vi "UHR-Fleezers Control (host) - 10.8MV_trial.vi"() -> ()   [LabVIEW 2010] (continued)
          }
          frame #2 {
            n1089 = property on="Green Laser ON/Interlacing" class="Bool (strict)"("Val(Sgnl)"=TRUE ("Value (Signaling)")) -> ()  [unwired: 2 in, 2 out]
            n1090 = property on="Flip Green Filter" class="Bool (strict)"("Val(Sgnl)"=TRUE ("Value (Signaling)")) -> ()  [unwired: 2 in, 2 out]
            n1091 = property on="Green laser mode" class="RadioBtnsControl (strict)"("Val(Sgnl)"=enum32{"Laser ON", "Laser OFF", "Interlace"}."Laser ON" ("Value (Signaling)")) -> ()  [unwired: 2 in, 2 out]
          }
          frame #3 {
            n1092 = Wait (ms)(milliseconds to wait=u32 500) -> ()  [unwired: 1 out]
          }
          frame #4 {
            n1093 = property on="Confocal Image" class="Bool (strict)"("Val(Sgnl)"=TRUE ("Value (Signaling)")) -> ()  [unwired: 2 in, 2 out]
          }
          frame #5 {
            n1094 = Wait (ms)(milliseconds to wait=u32 2000) -> ()  [unwired: 1 out]
          }
          frame #6 {
            n1095 = while {
              stop <- w5166 stop-if-true
              n1096 = local read "Saving..."() -> (w5167:bool)
              n1097 = Not(x=w5167) -> (.not. x?=w5166:bool)
            }
          }
          frame #7 {
            n1098 = property on="Flip Green Filter" class="Bool (strict)"("Val(Sgnl)"=TRUE ("Value (Signaling)")) -> ()  [unwired: 2 in, 2 out]
            n1099 = property on="Green Laser ON/Interlacing" class="Bool (strict)"("Val(Sgnl)"=w5171) -> ()  [unwired: 2 in, 2 out]
            n1100 = property on="Green laser mode" class="RadioBtnsControl (strict)"("Val(Sgnl)"=w5170) -> ()  [unwired: 2 in, 2 out]
          }
          frame #8 {
            n1101 = property on="Green FB On/Off" class="Bool (strict)"("Val(Sgnl)"=w5172) -> ()  [unwired: 2 in, 2 out]
          }
        }
      }
      event "Stop All": Value Change {
        n1102 = event-data() -> ()  [unwired: 1 in, 5 out]
        n1103 = local read "Stop All"() -> (w5173:bool)
      }
    }
    n1104 = node-c288() -> ()  [unwired: 1 in, 1 out]
  }
  n1105 = node-c288() -> (w76:T26)  [unwired: 4 out]
  n1106 = timed-loop "Mouse control: trap position (AOM deflection), set confocal spot from image" {
    tunnel: [w5175] -> w34
    tunnel: w24 -> [w5174]
    timing: w76 -> [_]
    timing-out: [_] -> w75
    stop <- w5175 stop-if-true
    n1107 = node-c288() -> ()  [unwired: 2 out]
    n1108 = event shown="[0] \"Pane\": Mouse Down" {
      selector: _ -> [_ _]
      dyn-events: _ -> [_ _]
      timeout: _ -> [_ _]
      tunnel: w5174 -> [w5178 _]
      event Mouse Down {
        n1109 = event-data() -> ("Time"=w5180:u32, "Coords"=w5179:T7, "Button"=w5181:u16)  [unwired: 6 out]
        n1110 = case shown="1" w5181 {
          tunnel: w5180 -> [_ _ w5284]
          tunnel: w5179 -> [_ w5218 w5282]
          tunnel: w5178 -> [_ _ w5280]
          frame 0, Default {
          }
          frame 1 {
            n1111 = property on="APD 2" class="ImageControl"() -> ("Displayed Image Position"=w5188:cluster{"Left":i32, "Top":i32})  [unwired: 2 in, 2 out]
            n1112 = property on="APD 1" class="ImageControl"() -> ("Displayed Image Position"=w5217:cluster{"Left":i32, "Top":i32})  [unwired: 2 in, 2 out]
            n1113 = property on="Detection Laser X" class="ImageControl"() -> ("Displayed Image Position"=w5214:cluster{"Left":i32, "Top":i32})  [unwired: 2 in, 2 out]
            n1114 = property on="Detection Laser Y" class="ImageControl"() -> ("Displayed Image Position"=w5213:cluster{"Left":i32, "Top":i32})  [unwired: 2 in, 2 out]
            n1115 = property on="APD 2" class="ImageControl"() -> ("Displayed Image Size"=w5187:cluster{"Width":u32, "Height":u32})  [unwired: 2 in, 2 out]
            n1116 = property on="APD 1" class="ImageControl"() -> ("Displayed Image Size"=w5215:cluster{"Width":u32, "Height":u32})  [unwired: 2 in, 2 out]
            n1117 = property on="Detection Laser X" class="ImageControl"() -> ("Displayed Image Size"=w5216:cluster{"Width":u32, "Height":u32})  [unwired: 2 in, 2 out]
            n1118 = property on="Detection Laser Y" class="ImageControl"() -> ("Displayed Image Size"=w5212:cluster{"Width":u32, "Height":u32})  [unwired: 2 in, 2 out]
            n1119 = Unbundle By Name(w5187) -> ("Width"=w5184:u32, "Height"=w5183:u32)
            n1120 = Unbundle By Name(w5188) -> ("Left"=w5186:i32, "Top"=w5185:i32)
            n1121 = Unbundle By Name(w5215) -> ("Width"=w5209:u32, "Height"=w5208:u32)
            n1122 = Unbundle By Name(w5216) -> ("Width"=w5205:u32, "Height"=w5204:u32)
            n1123 = Unbundle By Name(w5212) -> ("Width"=w5201:u32, "Height"=w5200:u32)
            n1124 = Unbundle By Name(w5217) -> ("Left"=w5211:i32, "Top"=w5210:i32)
            n1125 = Unbundle By Name(w5214) -> ("Left"=w5207:i32, "Top"=w5206:i32)
            n1126 = Unbundle By Name(w5213) -> ("Left"=w5203:i32, "Top"=w5202:i32)
            n1127 = Bundle("Left"=w5186, "Top"=w5185, "Width"=w5184, "Height"=w5183) -> (w5182:T35)  [unwired: 1 in]
            n1128 = Bundle("Left"=w5211, "Top"=w5210, "Width"=w5209, "Height"=w5208) -> (w5199:T35)  [unwired: 1 in]
            n1129 = Bundle("Left"=w5207, "Top"=w5206, "Width"=w5205, "Height"=w5204) -> (w5198:T35)  [unwired: 1 in]
            n1130 = Bundle("Left"=w5203, "Top"=w5202, "Width"=w5201, "Height"=w5200) -> (w5197:T35)  [unwired: 1 in]
            n1131 = Build Cluster Array(w5182, w5199, w5198, w5197) -> (w5196:T36)
            n1132 = for {
              tunnel: w5218 -> [w5229]
              tunnel: w5196 -> [w5230] mode=indexing
              shift-right: [w5227] -> w5194
              shift-left: TRUE -> [w5228]
              shift-right: [w5226] -> w5192
              shift-left: _ -> [w5222]
              shift-right: [w5225] -> w5191
              shift-left: _ -> [w5221]
              shift-right: [w5224] -> w5190
              shift-left: _ -> [w5220]
              shift-right: [w5223] -> w5189
              shift-left: _ -> [w5219]
              n1133 = case shown="True" w5228 {
                selector: w5228 -> [w5235 _]
                tunnel: w5230 -> [_ w5244]
                tunnel: w5229 -> [_ w5242]
                tunnel: [w5235 w5240] -> w5227
                tunnel: [w5234 w5239] -> w5226
                tunnel: [w5233 w5238] -> w5225
                tunnel: [w5232 w5237] -> w5224
                tunnel: [w5231 w5236] -> w5223
                tunnel: w5222 -> [w5234 _]
                tunnel: w5221 -> [w5233 _]
                tunnel: w5220 -> [w5232 _]
                tunnel: w5219 -> [w5231 _]
                frame False {
                }
                frame True {
                  n1134 = Unbundle(w5244) -> (w5243:T35)
                  n1135 = call "isclickinwindow.vi"("Image Param"=w5243, "Point32"=w5242) -> ("4 Y"=w5236:i32, "3 Height"=w5237:i32, "2 X"=w5238:i32, "1 Width"=w5239:i32, "In image?"=w5241:bool)  [unwired: 1 in]
                  n1136 = Not(x=w5241) -> (.not. x?=w5240:bool)
                }
              }
            }
            n1137 = Not(x=w5194) -> (.not. x?=w5193:bool)
            n1138 = case shown="True" w5193 {
              tunnel: w5191 -> [_ w5257]
              tunnel: w5189 -> [_ w5256]
              tunnel: w5192 -> [_ w5255]
              tunnel: w5190 -> [_ w5254]
              frame False {
              }
              frame True {
                w5250 = FALSE ("Get Point")
                n1139 = local read "Scan lines (y)"() -> (w5259:u64)
                n1140 = local read "Actual MCL Inc (V)"() -> (w5251:dbl)
                n1141 = local read "Scan steps (MCL)"() -> (w5258:u64)
                n1142 = Divide "Y Pix/step"(x=w5254, y=w5259) -> (x/y=w5266:dbl)
                n1143 = Divide "Y V/pix"(x=w5251, y=w5266) -> (x/y=w5265:dbl)
                n1144 = Divide "Y half step offset"(x=w5251, y=2.0) -> (x/y=w5267:dbl)
                n1145 = Divide "X pix/step"(x=w5255, y=w5258) -> (x/y=w5264:dbl)
                n1146 = Negate(x=w5267) -> (-x=w5268:dbl)
                n1147 = local read "Initial Y"() -> (w5274:dbl)
                n1148 = Multiply(x=w5256, y=w5265) -> (x*y=w5275:dbl)
                n1149 = Divide "X half step offset"(x=w5251, y=2.0) -> (x/y=w5261:dbl)
                n1150 = Divide "X V/pix"(x=w5251, y=w5264) -> (x/y=w5263:dbl)
                n1151 = Multiply(x=w5251, y=w5258) -> (x*y=w5270:dbl)
                n1152 = Compound Arithmetic op=ADD(w5268, w5275, w5274) -> (w5252:dbl)
                "Pointer Y (V)" <- w5252
                n1153 = Multiply(x=w5263, y=w5257) -> (x*y=w5272:dbl)
                n1154 = Negate(x=w5261) -> (-x=w5260:dbl)
                n1155 = local read "Initial X"() -> (w5273:dbl)
                n1156 = Negate(x=w5272) -> (-x=w5271:dbl)
                n1157 = Compound Arithmetic op=ADD(w5260, w5270, w5273, w5271) -> (w5253:dbl)
                "Pointer X (V)" <- w5253
                n1158 = Or(x="Set X Only", y="Set Confocal Spot (X-Y)") -> (x .or. y?=w5246:bool)
                n1159 = Or(x="Set Confocal Spot (X-Y)", y="Set Y Only") -> (x .or. y?=w5245:bool)
                n1160 = case shown="True" w5246 {
                  tunnel: w5253 -> [_ w5276]
                  frame False {
                  }
                  frame True {
                    n1161 = property on="AO2" class="Slide (strict)"("Val(Sgnl)"=w5276) -> ()  [unwired: 2 in, 2 out]
                  }
                }
                n1162 = case shown="True" w5245 {
                  tunnel: w5252 -> [_ w5277]
                  frame False {
                  }
                  frame True {
                    n1163 = property on="AO1" class="Slide (strict)"("Val(Sgnl)"=w5277) -> ()  [unwired: 2 in, 2 out]
                  }
                }
                n1164 = local write "Set Confocal Spot (X-Y)"(w5250) -> ()
                n1165 = local write "Set X Only"(w5250) -> ()
                n1166 = local write "Set Y Only"(w5250) -> ()
              }
            }
          }
          frame 3 {
            n1167 = local read "BD 2 Frequency 1 (MHz)"() -> (w5278:dbl)
            n1168 = local read "BD 1 Frequency 1 (MHz)"() -> (w5279:dbl)
            n1169 = local write "Manipulating Trap"(TRUE ("Manipulating Trap")) -> ()
            n1170 = local write "Coords"(T7 {"Horizontal"=0, "Vertical"=0} ("Coords")) -> ()
            n1171 = while {
              tunnel: w5284 -> [w5289]
              tunnel: w5282 -> [w5288]
              tunnel: w5280 -> [w5287]
              tunnel: w5279 -> [w5286]
              tunnel: w5278 -> [w5285]
              stop <- w5290 stop-if-true
              n1172 = event shown="[0] \"Pane\": Mouse Move" {
                selector: _ -> [_ _]
                dyn-events: _ -> [_ _]
                timeout: _ -> [_ _]
                tunnel: ["Force Manip Abort" w5354] -> w5290
                tunnel: w5289 -> [w5297 _]
                tunnel: w5288 -> [w5295 _]
                tunnel: w5287 -> [w5294 _]
                tunnel: w5286 -> [w5293 _]
                tunnel: w5285 -> [w5292 _]
                event Mouse Move {
                  n1173 = event-data() -> ("Time"=w5298:u32, "Coords"=w5299:T7)  [unwired: 3 out]
                  n1174 = Less?(x=w5298, y=w5297) -> (x < y?=w5296:bool)
                  n1175 = case "Makes sure old motion events prior to mouse click aren't used" shown="False" w5296 {
                    tunnel: w5299 -> [w5341 _]
                    tunnel: w5295 -> [w5342 _]
                    tunnel: w5294 -> [w5319 _]
                    tunnel: w5293 -> [w5315 _]
                    tunnel: w5292 -> [w5314 _]
                    frame False {
                      n1176 = Subtract(x=w5341, y=w5342) -> (x-y=w5340:T7)
                      "Coords" <- w5340
                      n1177 = local read "Y RF Frequency Limits (MHz)"() -> (w5300:T16)
                      n1178 = To Double Precision Float(number=w5340) -> (double precision float=w5339:cluster{"Horizontal":dbl, "Vertical":dbl})
                      n1179 = Multiply(x=cluster{"Horizontal":dbl, "Vertical":dbl} {"Horizontal"=-1.0, "Vertical"=1.0}, y="Manipulation Scaling") -> (x*y=w5335:cluster{"Horizontal":dbl, "Vertical":dbl})
                      n1180 = local read "X RF Frequency Limits (MHz)"() -> (w5301:T16)
                      n1181 = Multiply(x=w5339, y=w5335) -> (x*y=w5337:cluster{"Horizontal":dbl, "Vertical":dbl})
                      n1182 = Unbundle By Name(w5337) -> ("Horizontal"=w5332:dbl, "Vertical"=w5336:dbl)
                      n1183 = Unbundle By Name(w5300) -> ("Maximum"=w5303:dbl, "Minimum"=w5302:dbl)
                      n1184 = Boolean To (0,1)(Boolean="Manip. X?") -> (0, 1=w5330:i16)
                      n1185 = Boolean To (0,1)(Boolean="Manip. Y?") -> (0, 1=w5327:i16)
                      n1186 = local read "BD 1 Frequency 2 (MHz)"() -> (w5317:dbl)
                      n1187 = Multiply(x=w5336, y=w5327) -> (x*y=w5329:dbl)
                      n1188 = Multiply(x=w5330, y=w5332) -> (x*y=w5333:dbl)
                      n1189 = local read "BD 2 Frequency 2 (MHz)"() -> (w5316:dbl)
                      n1190 = Unbundle By Name(w5301) -> ("Maximum"=w5305:dbl, "Minimum"=w5304:dbl)
                      n1191 = Add(x=w5314, y=w5329) -> (x+y=w5307:dbl)
                      n1192 = Add(x=w5315, y=w5333) -> (x+y=w5309:dbl)
                      n1193 = In Range and Coerce(upper limit=w5305, x=w5309, lower limit=w5304) -> (coerced(x)=w5308:dbl)  [unwired: 1 out]
                      n1194 = In Range and Coerce(upper limit=w5303, x=w5307, lower limit=w5302) -> (coerced(x)=w5306:dbl)  [unwired: 1 out]
                      n1195 = Subtract(x=w5308, y=w5317) -> (x-y=w5326:dbl)
                      n1196 = Subtract(x=w5306, y=w5316) -> (x-y=w5325:dbl)
                      n1197 = Square(x=w5326) -> (x^2=w5324:dbl)
                      n1198 = Square(x=w5325) -> (x^2=w5323:dbl)
                      n1199 = Add(x=w5324, y=w5323) -> (x+y=w5322:dbl)
                      n1200 = Square Root(x=w5322) -> (sqrt(x)=w5318:dbl)
                      n1201 = In Range and Coerce(upper limit="Limit Max (MHz)", x=w5318, lower limit="Limit Min (MHz)") -> (In Range?=w5311:bool)  [unwired: 1 out]
                      n1202 = Not(x="Limits Enable") -> (.not. x?=w5310:bool)
                      n1203 = Or(x=w5311, y=w5310) -> (x .or. y?=w5312:bool)
                      n1204 = case shown="True" w5312 {
                        tunnel: w5319 -> [_ w5352]
                        tunnel: w5318 -> [_ w5343]
                        tunnel: w5308 -> [_ w5350]
                        tunnel: w5317 -> [_ w5349]
                        tunnel: w5306 -> [_ w5348]
                        tunnel: w5316 -> [_ w5347]
                        tunnel: w5301 -> [_ w5345]
                        tunnel: w5300 -> [_ w5344]
                        frame False {
                        }
                        frame True {
                          n1205 = local read "BD 1 Frequency 3 (MHz)"() -> (w5351:dbl)
                          n1206 = local read "BD 2 Frequency 3 (MHz)"() -> (w5346:dbl)
                          n1207 = local write "Trap Delta (MHz)"(w5343) -> ()
                          n1208 = property on="Initial delta (MHz)" class="DigNum (strict)"("Val(Sgnl)"=w5343) -> ()  [unwired: 2 in, 2 out]
                          n1209 = call "set RF board frequency - interlace.vi"("Board 2 Frequency Limits"=w5344, "Board 1 Frequency Limits"=w5345, "FPGA VI Reference In"=w5352, "Board 2 Frequency 3 (MHz)"=w5346, "Board 1 Frequency 3 (MHz)"=w5351, "Board 2 Frequency 2 (MHz)"=w5347, "Board 2 Frequency 1 (MHz)"=w5348, "Board 1 Frequency 2 (MHz)"=w5349, "Board 1 Frequency 1  (MHz)"=w5350) -> ()  [unwired: 1 in, 2 out]
                          n1210 = local write "BD 2 Frequency 1 (MHz)"(w5348) -> ()
                          n1211 = local write "BD 1 Frequency 1 (MHz)"(w5350) -> ()
                        }
                      }
                    }
                    frame True {
                    }
                  }
                }
                event Mouse Up {
                  n1212 = event-data() -> ("Button"=w5353:u16)  [unwired: 8 out]
                  n1213 = case shown="3" w5353 {
                    tunnel: [FALSE TRUE] -> w5354
                    frame 0, Default {
                    }
                    frame 3 {
                      n1214 = local write "Manipulating Trap"(FALSE ("Manipulating Trap")) -> ()
                    }
                  }
                }
              }
            }
          }
        }
      }
      event Mouse Move {
        n1215 = event-data() -> ()  [unwired: 6 out]
      }
    }
    n1216 = local read "Stop All"() -> (w5175:bool)
    n1217 = node-c288() -> ()  [unwired: 2 out]
  }
  n1218 = node-c288(i64 1 ("Period"), 1 ("Processor")) -> (w164:T26)  [unwired: 2 out]
  n1219 = timed-loop "Acquire Data" {
    tunnel: w24 -> [w5612]
    tunnel: w40 -> [w5611]
    tunnel: [w5642] -> w33
    tunnel: [w5636] -> w32
    timing: w164 -> [_]
    timing-out: [_] -> w163
    tunnel: w59 -> [w5440]
    stop <- "Stop All" stop-if-true
    (unwired) u32 0 ("Number of Elements")
    w5427 = "NI_ChannelName" ("name")
    n1220 = node-c288() -> ()  [unwired: 2 out]
    n1221 = First Call?() -> (First Call?: T/F=w5393:bool)
    n1222 = Or(x="Reset", y=w5393) -> (x .or. y?=w5394:bool)
    n1223 = case "Reset data stream" shown="True" w5394 {
      tunnel: w5612 -> [w5730 w5738]
      tunnel: w5611 -> [w5729 w5737]
      tunnel: [w5730 w5732] -> w5607
      tunnel: [w5729 w5731] -> w5606
      frame False {
      }
      frame True {
        w5735 = TRUE ("AI to FIFO")
        n1224 = local write "Overflow (data lost)"(FALSE ("Overflow (data lost)")) -> ()
        n1225 = call "reset FPGA DMA.vi"("error in"=w5737, "FPGA VI Reference In"=w5738) -> ("error out"=w5733:errorcluster, "FPGA VI Reference Out"=w5734:T19)
        n1226 = xnode "Read/Write Control"("FPGA VI Reference In"=w5734, "error in"=w5733, "AI to FIFO"=w5735, "APD to FIFO"=w5735) -> ("FPGA VI Reference Out"=w5732:T19, "error out"=w5731:errorcluster)
      }
    }
    n1227 = Or(x="Start AOD Scan", y="Trap Raster Scan") -> (x .or. y?=w5557:bool)
    n1228 = case "Start AOM raster scan" shown="True" w5557 {
      tunnel: w5607 -> [w7338 w7348]
      tunnel: w5606 -> [w7337 w7347]
      tunnel: [w7338 w7341] -> w5605
      tunnel: [w7337 w7340] -> w5604
      frame False {
      }
      frame True {
        n1229 = case shown="True" "Restart DMA? (AOD)" {
          tunnel: [w7759 w7761] -> w7342
          tunnel: [w7758 w7760] -> w7343
          tunnel: w7348 -> [w7759 w7763]
          tunnel: w7347 -> [w7758 w7762]
          frame False {
          }
          frame True {
            n1230 = local write "Overflow (data lost)"(FALSE ("Overflow (data lost)")) -> ()
            n1231 = call "reset FPGA DMA.vi"("error in"=w7762, "FPGA VI Reference In"=w7763) -> ("error out"=w7760:errorcluster, "FPGA VI Reference Out"=w7761:T19)
          }
        }
        n1232 = local write "Trap Raster Scan"(FALSE ("Trap Raster Scan")) -> ()
        n1233 = case shown="False" "Move MCL Also?" {
          tunnel: w7343 -> [w7351 w7460]
          tunnel: w7342 -> [w7352 w7461]
          tunnel: [w7350 w7464] -> w7341
          tunnel: [w7349 w7463] -> w7340
          frame False {
            w7353 = TRUE ("AI to FIFO")
            n1234 = xnode "Read/Write Control"("FPGA VI Reference In"=w7352, "error in"=w7351, "AI to FIFO"=w7353, "APD to FIFO"=w7353, "Start scan"=w7353) -> ("FPGA VI Reference Out"=w7350:T19, "error out"=w7349:errorcluster)
          }
          frame True {
            w7457 = FALSE ("1D or 2D Scan?")
            w7462 = TRUE ("AI to FIFO")
            # "Count for MCL loop"
            # "N total cycles"
            # "N steps"
            # "V_int"
            n1235 = local read "Scan Range (nm)"() -> (w7439:dbl)
            n1236 = local read "Number of F/B Scans (AOD)"() -> (w7456:u16)
            n1237 = Sign(1:w7439) -> (0:w7438:dbl)
            n1238 = Compound Arithmetic op=MULTIPLY(w7439, "MCL Step Position Ratio", "MCL/AOM Scale Tweak") -> (w7443:dbl)
            n1239 = Negate(x=w7438) -> (-x=w7435:dbl)
            n1240 = Multiply(x=w7435, y="MCL Step Increment (V_int)") -> (x*y=w7437:dbl)
            n1241 = Divide(x=w7443, y="MCL X Cal (nm/V)") -> (x/y=w7449:dbl)
            n1242 = Multiply(x=32767.0 ("y"), y=w7449) -> (x*y=w7455:dbl)
            n1243 = local read "Total Counts (ticks)"() -> (w7440:u32)
            n1244 = local read "Cycles/step (AOD)"() -> (w7451:u64)
            n1245 = local read "Scan steps (AOD)"() -> (w7452:u64)
            n1246 = Divide(x=w7455, y=10.0) -> (x/y=w7448:dbl)
            n1247 = Divide(x=w7448, y="MCL Step Increment (V_int)") -> (x/y=w7446:dbl)
            n1248 = Absolute Value(x=w7446) -> (abs(x)=w7434:dbl)
            n1249 = Compound Arithmetic op=MULTIPLY(w7452, w7451, w7440) -> (w7447:u64)
            n1250 = local write "wait to reset values"(w7462) -> ()
            n1251 = local write "MCL Scanning"(w7462) -> ()
            n1252 = Divide(x=w7447, y=w7434) -> (x/y=w7444:dbl)
            "MCL Count" <- w7444
            n1253 = xnode "Read/Write Control"("FPGA VI Reference In"=w7461, "error in"=w7460, "Scan steps (MCL)"=w7434, "Number of scans (MCL)"=w7456, "Cycles per step (MCL)"=u64 1, "Scan freq.  increment (MCL)"=w7437, "1D or 2D Scan?"=w7457, "MCL Scan Axis"=w7457, "Cont. Scan (MCL)"=w7457, "MCL count"=w7444) -> ("FPGA VI Reference Out"=w7459:T19, "error out"=w7458:errorcluster)
            n1254 = xnode "Read/Write Control"("FPGA VI Reference In"=w7459, "error in"=w7458, "AI to FIFO"=w7462, "APD to FIFO"=w7462, "Start scan"=w7462, "Start scan (MCL)"=w7462) -> ("FPGA VI Reference Out"=w7464:T19, "error out"=w7463:errorcluster)
          }
        }
        "Raster Scanning..." <- TRUE ("Scanning...")
      }
    }
    n1255 = And(x="Save scans", y=w5557) -> (x .and. y?=w5603:bool)
    n1256 = Compound Arithmetic op=OR("Start MCL Scan", "Confocal Image", "Confocal Linescan") -> (w5555:bool)
    n1257 = And(x="Save Data (MCL)", y=w5555) -> (x .and. y?=w5602:bool)
    n1258 = case "Start MCL raster scan" shown="True" w5555 {
      tunnel: w5605 -> [w6615 w6630]
      tunnel: w5604 -> [w6614 w6629]
      tunnel: [w6615 w6625] -> w5362
      tunnel: [w6614 w6624] -> w5361
      tunnel: [FALSE w6623] -> w5588
      tunnel: "Start MCL Scan" -> [_ w6618]
      tunnel: "Confocal Image" -> [_ w6617]
      tunnel: "Confocal Linescan" -> [_ _]
      frame False {
      }
      frame True {
        w6623 = TRUE
        n1259 = case shown="True" "Restart DMA? (MCL)" {
          tunnel: [w6875 w6877] -> w6628
          tunnel: [w6874 w6876] -> w6627
          tunnel: w6630 -> [w6875 w6880]
          tunnel: w6629 -> [w6874 w6879]
          frame False {
          }
          frame True {
            n1260 = call "reset FPGA DMA.vi"("error in"=w6879, "FPGA VI Reference In"=w6880) -> ("error out"=w6876:errorcluster, "FPGA VI Reference Out"=w6877:T19)
            n1261 = local write "Overflow (data lost)"(FALSE ("Overflow (data lost)")) -> ()
          }
        }
        n1262 = case shown="False" w6618 {
          selector: w6618 -> [_ w6634]
          tunnel: w6617 -> [w6633 _]
          tunnel: [w6633 w6634] -> w6616
          frame False {
            n1263 = property on="2D or 1D Scan" class="Bool (strict)"("Val(Sgnl)"=w6633) -> ()  [unwired: 2 in, 2 out]
            n1264 = property on="Confocal Image" class="Bool (strict)"("Value"=FALSE ("Start Confocal Map")) -> ()  [unwired: 2 in, 2 out]
          }
          frame True {
          }
        }
        n1265 = local write "MCL Scanning"(w6623) -> ()
        n1266 = local read "AO1"() -> (w6620:dbl)
        n1267 = local read "AO2"() -> (w6619:dbl)
        n1268 = case shown="True" "Center Scan" {
          tunnel: w6628 -> [w6641 w6753]
          tunnel: w6627 -> [w6640 w6752]
          tunnel: [w6639 w6751] -> w6625
          tunnel: [w6638 w6750] -> w6624
          tunnel: [w6636 w6737] -> w6622
          tunnel: [w6635 w6736] -> w6621
          tunnel: w6620 -> [w6636 w6742]
          tunnel: w6619 -> [w6635 w6745]
          tunnel: w6616 -> [_ _]
          frame False {
            w6637 = TRUE ("AI to FIFO")
            n1269 = xnode "Read/Write Control"("FPGA VI Reference In"=w6641, "error in"=w6640, "AI to FIFO"=w6637, "APD to FIFO"=w6637, "Start scan (MCL)"=w6637) -> ("FPGA VI Reference Out"=w6639:T19, "error out"=w6638:errorcluster)
          }
          frame True {
            w6749 = TRUE ("AI to FIFO")
            n1270 = local read "Scan steps (MCL)"() -> (w6728:u64)
            n1271 = local read "Scan lines (y)"() -> (w6724:u64)
            n1272 = local read "Fast Scan Dir"() -> (w6735:bool)
            n1273 = local read "Actual MCL Inc (V)"() -> (w6725:dbl)
            n1274 = Decrement(x=w6724) -> (x-1=w6723:u64)
            n1275 = Decrement(x=w6728) -> (x-1=w6727:u64)
            n1276 = Multiply(x=w6725, y=w6723) -> (x*y=w6722:dbl)
            n1277 = Divide(x=w6722, y=2.0) -> (x/y=w6732:dbl)
            n1278 = Multiply(x=w6725, y=w6727) -> (x*y=w6726:dbl)
            n1279 = Divide(x=w6726, y=2.0) -> (x/y=w6731:dbl)
            n1280 = Select(t=w6731, s=w6735, f=w6732) -> (s? t:f=w6730:dbl)
            n1281 = Select(t=w6732, s=w6735, f=w6731) -> (s? t:f=w6734:dbl)
            n1282 = Subtract(x=w6742, y=w6734) -> (x-y=w6733:dbl)
            n1283 = Subtract(x=w6745, y=w6730) -> (x-y=w6729:dbl)
            n1284 = local read "2D or 1D Scan"() -> (w6747:bool)
            n1285 = Not(x=w6735) -> (.not. x?=w6741:bool)
            n1286 = Not(x=w6747) -> (.not. x?=w6743:bool)
            n1287 = And(x=w6735, y=w6743) -> (x .and. y?=w6744:bool)
            n1288 = And(x=w6743, y=w6741) -> (x .and. y?=w6746:bool)
            n1289 = Select(t=w6745, s=w6746, f=w6729) -> (s? t:f=w6736:dbl)
            n1290 = Select(t=w6742, s=w6744, f=w6733) -> (s? t:f=w6737:dbl)
            n1291 = call "Volt to I16.vi"("Voltage In"=w6737) -> ("I16 Voltage Out"=w6740:i16)
            n1292 = call "Volt to I16.vi"("Voltage In"=w6736) -> ("I16 Voltage Out"=w6739:i16)
            n1293 = xnode "Read/Write Control"("FPGA VI Reference In"=w6753, "error in"=w6752, "AI to FIFO"=w6749, "APD to FIFO"=w6749, "Start scan (MCL)"=w6749, "AO1"=w6740, "AO2"=w6739) -> ("FPGA VI Reference Out"=w6751:T19, "error out"=w6750:errorcluster)
          }
        }
        "Initial Y" <- w6622
        "Initial X" <- w6621
        "wait to reset values" <- w6623
      }
    }
    n1294 = local read "Trap Pos Elements/DMA read"() -> (w5436:u32)
    n1295 = local read "Trap AI Elements/DMA read"() -> (w5360:u32)
    n1296 = local read "APD Elements/DMA read"() -> (w5479:u32)
    n1297 = local read "Trap AI FIFO Depth"() -> (w5652:u32)
    n1298 = xnode "Invoke Method"("FPGA VI Reference In"=w5362, "error in"=w5361, "Number of Elements"=w5436, "Timeout (ms)"=-1) -> ("Data"=w5400:u16[], "Elements Remaining"=→"Trap Pos FIFO El Remaining":u32)  [unwired: 2 out]
    n1299 = xnode "Invoke Method"("FPGA VI Reference In"=w5362, "error in"=w5361, "Number of Elements"=w5360, "Timeout (ms)"=-1 ("Timeout")) -> ("FPGA VI Reference Out"=w5364:T19, "error out"=w5363:errorcluster, "Data"=w5359:i16[], "Elements Remaining"=w5365:u32)
    "Trap AI FIFO El. Rem." <- w5365
    n1300 = xnode "Get APD Data"("FPGA VI Reference In"=w5362, "error in"=w5361, "Number of Elements"=w5479, "Timeout (ms)"=-1) -> ("Data"=w5478:u32[], "Elements Remaining"=→"APD FIFO Elements Remaining":u32)  [unwired: 2 out]
    n1301 = Subtract(x=w5652, y=w5360) -> (x-y=w5651:u32)
    n1302 = Decimate 1D Array(w5400) -> (w5397:u16[], w5399:u16[], w5398:u16[])
    n1303 = Divide(x=w5365, y=w5651) -> (x/y=w5650:dbl)
    "Buffer Status" <- w5650
    n1304 = To Unsigned Long Integer(number=w5397) -> (unsigned 32bit integer=w5396:u32[])
    n1305 = Join Numbers(hi=w5399, lo=w5398) -> ((hi.lo)=w5395:u32[])
    n1306 = Equal?(x=w5650, y=1.0) -> (x = y?=w5648:bool)
    n1307 = Join Numbers(hi=w5396, lo=w5395) -> ((hi.lo)=w5389:u64[])
    n1308 = call "IR AOM word to freq - vec.vi"("Frequency Word In (double vec)"=w5389) -> ("Frequency Out"=w5435:dbl[])
    n1309 = case "Alert buffer overflow" shown="True" w5648 {
      frame False {
      }
      frame True {
        n1310 = call <vilib>:"Beep.vi"() -> ()  [unwired: 3 in, 9 out]
        "Overflow (data lost)" <- TRUE ("Overflow (data lost)")
      }
    }
    n1311 = Decimate 1D Array(w5435) -> (w5434:dbl[], w5433:dbl[])
    n1312 = Array Size(array=w5359) -> (size(s)=→"Waveform Chart":i32)
    n1313 = Build Array(w5434, w5433) -> (w5432:dbl[][])
    n1314 = local read "Trap Sets"() -> (w5516:u32)
    n1315 = case "Deinterlace trap data, average down PSD" shown="2" w5516 {
      tunnel: w5359 -> [w6910 w6975]
      tunnel: [w6907 w6972] -> w5509
      tunnel: [w6910 w6974] -> w5392
      tunnel: "Detector Type" -> [w6909 w6970]
      tunnel: [w6908 w6973] -> w5508
      tunnel: [w6906 w6971] -> w5623
      frame 1, Default {
        n1316 = Divide(x=w6910, y=3276.7) -> (x/y=w6911:dbl[])
        n1317 = Decimate 1D Array(w6911) -> (w6920:dbl[], w6919:dbl[], w6918:dbl[], w6917:dbl[], w6916:dbl[], w6915:dbl[], w6914:dbl[], w6913:dbl[])
        n1318 = case shown="\"IR-QPD + PSD + FB-QPD position\"" w6909 {
          tunnel: w6920 -> [w6944 w6969]
          tunnel: w6919 -> [w6943 w6968]
          tunnel: w6918 -> [w6928 w6946]
          tunnel: w6917 -> [w6929 w6956]
          tunnel: w6916 -> [w6942 w6967]
          tunnel: w6915 -> [w6941 w6966]
          tunnel: w6914 -> [w6925 w6947]
          tunnel: w6913 -> [w6924 w6945]
          tunnel: [w6923 w6953] -> w6908
          tunnel: [w6922 w6952] -> w6907
          tunnel: [w6921 w6951] -> w6906
          frame "IR-QPD + PSD + FB-QPD", Default {
            w6921 = 0  # Channel pattern
            n1319 = Divide(x=w6944, y=w6929) -> (x/y=w6931:dbl[])
            n1320 = Divide(x=w6943, y=w6929) -> (x/y=w6930:dbl[])
            n1321 = Divide(x=w6942, y=w6925) -> (x/y=w6927:dbl[])
            n1322 = Divide(x=w6941, y=w6924) -> (x/y=w6926:dbl[])
            n1323 = Build Array(w6931, w6930, w6929, w6928, w6927, w6926, w6925, w6924) -> (w6922:dbl[][])
            n1324 = Bundle("T1 Y", "T1 X", "T1 Sum", "FB Sum", "PSD Y", "PSD X", "PSD Y Sum", "PSD X Sum") -> (w6940:T44)  [unwired: 1 out]
            n1325 = Cluster To Array(cluster=w6940) -> (array=w6923:string[])
          }
          frame "IR-QPD + PSD + FB-QPD position" {
            w6951 = 3  # Channel pattern
            n1326 = Negate(x=w6947) -> (-x=w6948:dbl[])
            n1327 = Divide(x=w6969, y=w6956) -> (x/y=w6958:dbl[])
            n1328 = Divide(x=w6968, y=w6956) -> (x/y=w6957:dbl[])
            n1329 = Divide(x=w6967, y=w6947) -> (x/y=w6955:dbl[])
            n1330 = Divide(x=w6966, y=w6948) -> (x/y=w6954:dbl[])
            n1331 = Build Array(w6958, w6957, w6956, w6945, w6946, w6955, w6954, w6947) -> (w6952:dbl[][])
            n1332 = Bundle("T1 Y", "T1 X", "T1 Sum", "FB X", "FB Sum", "PSD Y", "PSD X", "PSD Y Sum") -> (w6965:T44)  [unwired: 1 out]
            n1333 = Cluster To Array(cluster=w6965) -> (array=w6953:string[])
          }
        }
      }
      frame 2 {
        n1334 = case shown="\"UCB Fleezers 052511\"" w6970 {
          tunnel: w6975 -> [w7037 w7104 w7132 w7239]
          tunnel: [w6976 w7096 w7127 w7170] -> w6974
          tunnel: [w7003 w7087 w7129 w7217] -> w6973
          tunnel: [w7002 w7051 w7106 w7184] -> w6972
          tunnel: [w6996 w7086 w7169 w7215] -> w6971
          frame "IR-QPD + PSD + FB-QPD", Default {
            w6996 = 1  # Channel pattern
            # "time average x2 the 4th signal and the 4 psd signals (detection laser)"
            # "deinterlace 3 signals from qpd"
            n1335 = Decimate 1D Array(w7037) -> (w7036:i16[], w7035:i16[], w7001:i16[], w7034:i16[], w7024:i16[], w7022:i16[], w7021:i16[], w7019:i16[])
            n1336 = call "downsample 1D array - double.vi"("Ave N"=2.0, "Array In"=w7024) -> ("Array Out"=w7023:dbl[])  [unwired: 1 out]
            n1337 = call "downsample 1D array - double.vi"("Ave N"=2.0, "Array In"=w7019) -> ("Array Out"=w7018:dbl[])  [unwired: 1 out]
            n1338 = call "downsample 1D array - double.vi"("Ave N"=2.0, "Array In"=w7021) -> ("Array Out"=w7020:dbl[])  [unwired: 1 out]
            n1339 = call "downsample 1D array - double.vi"("Ave N"=2.0, "Array In"=w7022) -> ("Array Out"=w7004:dbl[])  [unwired: 1 out]
            n1340 = Decimate 1D Array(w7036) -> (w7033:i16[], w7005:i16[])
            n1341 = Decimate 1D Array(w7035) -> (w7032:i16[], w7030:i16[])
            n1342 = Decimate 1D Array(w7034) -> (w7031:i16[], w7029:i16[])
            n1343 = Decimate 1D Array(w7001) -> (w7000:i16[], w6999:i16[])
            n1344 = Interleave 1D Arrays(w7033, w7032, w7031, w7005, w7030, w7029, w7000, w6999, w7023, w7004, w7020, w7018) -> (w7017:dbl[])
            n1345 = To Word Integer(number=w7017) -> (16bit integer=w6976:i16[])
            n1346 = Divide(x=w7017, y=3276.7) -> (x/y=w7016:dbl[])
            n1347 = Decimate 1D Array(w7016) -> (w7015:dbl[], w7014:dbl[], w7013:dbl[], w7012:dbl[], w7011:dbl[], w7010:dbl[], w6998:dbl[], w6997:dbl[], w7009:dbl[], w7008:dbl[], w7007:dbl[], w7006:dbl[])
            n1348 = Divide(x=w7015, y=w7013) -> (x/y=w6983:dbl[])
            n1349 = Divide(x=w7014, y=w7013) -> (x/y=w6982:dbl[])
            n1350 = Divide(x=w7012, y=w7010) -> (x/y=w6981:dbl[])
            n1351 = Divide(x=w7011, y=w7010) -> (x/y=w6980:dbl[])
            n1352 = Divide(x=w7009, y=w7007) -> (x/y=w6979:dbl[])
            n1353 = Divide(x=w7008, y=w7006) -> (x/y=w6978:dbl[])
            n1354 = Bundle("T1 Y", "T1 X", "T1 Sum", "T2 Y", "T2 X", "T2 Sum", "T1 FB Sum", "T2 FB Sum", "PSD Y", "PSD X", "PSD Y Sum", "PSD X Sum") -> (w6984:T45)  [unwired: 1 out]
            n1355 = Build Array(w6983, w6982, w7013, w6981, w6980, w7010, w6998, w6997, w6979, w6978, w7007, w7006) -> (w7002:dbl[][])
            n1356 = Cluster To Array(cluster=w6984) -> (array=w7003:string[])
          }
          frame "IR-QPD + PSD + FB-QPD X position" {
            w7086 = 2  # Channel pattern
            # "convert\nADC numbers\nto volts"
            # "time average x2 the 3 psd signals (detection laser)"
            # "deinterlace 3 signals from qpds"
            n1357 = Decimate 1D Array(w7104) -> (w7103:i16[], w7102:i16[], w7039:i16[], w7040:i16[], w7049:i16[], w7046:i16[], w7043:i16[], w7074:i16[])
            n1358 = Decimate 1D Array(w7103) -> (w7101:i16[], w7088:i16[])
            n1359 = call "downsample 1D array - I16.vi"("Ave N"=2.0, "Array In"=w7049) -> ("Array Out"=w7047:i16[])  [unwired: 1 in]
            n1360 = call "downsample 1D array - I16.vi"("Ave N"=2.0, "Array In"=w7046) -> ("Array Out"=w7044:i16[])  [unwired: 1 in]
            n1361 = Decimate 1D Array(w7102) -> (w7100:i16[], w7098:i16[])
            n1362 = Decimate 1D Array(w7040) -> (w7099:i16[], w7097:i16[])
            n1363 = Decimate 1D Array(w7074) -> (w7073:i16[], w7071:i16[])
            n1364 = Decimate 1D Array(w7039) -> (w7072:i16[], w7070:i16[])
            n1365 = call "downsample 1D array - I16.vi"("Ave N"=2.0, "Array In"=w7043) -> ("Array Out"=w7041:i16[])  [unwired: 1 in]
            n1366 = Interleave 1D Arrays(w7101, w7100, w7099, w7088, w7098, w7097, w7073, w7072, w7071, w7070, w7047, w7044, w7041) -> (w7096:i16[])
            n1367 = Divide(x=w7096, y=3276.7) -> (x/y=w7095:dbl[])
            n1368 = Decimate 1D Array(w7095) -> (w7094:dbl[], w7093:dbl[], w7092:dbl[], w7091:dbl[], w7090:dbl[], w7089:dbl[], w7062:dbl[], w7060:dbl[], w7059:dbl[], w7057:dbl[], w7056:dbl[], w7055:dbl[], w7052:dbl[])
            n1369 = Divide(x=w7094, y=w7092) -> (x/y=w7078:dbl[])
            n1370 = Divide(x=w7093, y=w7092) -> (x/y=w7077:dbl[])
            n1371 = Divide(x=w7091, y=w7089) -> (x/y=w7076:dbl[])
            n1372 = Divide(x=w7090, y=w7089) -> (x/y=w7075:dbl[])
            n1373 = Divide(x=w7062, y=w7060) -> (x/y=w7061:dbl[])
            n1374 = Divide(x=w7059, y=w7057) -> (x/y=w7058:dbl[])
            n1375 = Divide(x=w7056, y=w7052) -> (x/y=w7054:dbl[])
            n1376 = Negate(x=w7052) -> (-x=w7050:dbl[])
            n1377 = Divide(x=w7055, y=w7050) -> (x/y=w7053:dbl[])
            n1378 = Bundle("T1 Y", "T1 X", "T1 Sum", "T2 Y", "T2 X", "T2 Sum", "T1 FB X", "T1 FB Sum", "T2 FB X", "T2 FB Sum", "PSD Y", "PSD X", "PSD Y Sum") -> (w7079:T46)  [unwired: 1 out]
            n1379 = Build Array(w7078, w7077, w7092, w7076, w7075, w7089, w7061, w7060, w7058, w7057, w7054, w7053, w7052) -> (w7051:dbl[][])
            n1380 = Cluster To Array(cluster=w7079) -> (array=w7087:string[])
          }
          frame "UCB Fleezers 052511" {
            w7169 = 2  # Channel pattern
            n1381 = Decimate 1D Array(w7132) -> (w7167:i16[], w7166:i16[], w7131:i16[], w7130:i16[], w7124:i16[], w7121:i16[], w7120:i16[], w7119:i16[])
            n1382 = Decimate 1D Array(w7167) -> (w7165:i16[], w7150:i16[])
            n1383 = Decimate 1D Array(w7166) -> (w7164:i16[], w7162:i16[])
            n1384 = Decimate 1D Array(w7131) -> (w7163:i16[], w7161:i16[])
            n1385 = Decimate 1D Array(w7130) -> (w7126:i16[], w7125:i16[])
            n1386 = Decimate 1D Array(w7124) -> (w7123:i16[], w7122:i16[])
            n1387 = call "downsample 1D array - I16.vi"("Ave N"=2.0, "Array In"=w7121) -> ("Array Out"=w7118:i16[])  [unwired: 1 in]
            n1388 = call "downsample 1D array - I16.vi"("Ave N"=2.0, "Array In"=w7120) -> ("Array Out"=w7117:i16[])  [unwired: 1 in]
            n1389 = call "downsample 1D array - I16.vi"("Ave N"=2.0, "Array In"=w7119) -> ("Array Out"=w7116:i16[])  [unwired: 1 in]
            n1390 = Interleave 1D Arrays(w7165, w7164, w7163, w7150, w7162, w7161, w7126, w7123, w7125, w7122, w7118, w7117, w7116) -> (w7127:i16[])
            n1391 = Divide(x=w7127, y=3276.7) -> (x/y=w7157:dbl[])
            n1392 = Decimate 1D Array(w7157) -> (w7156:dbl[], w7155:dbl[], w7154:dbl[], w7153:dbl[], w7152:dbl[], w7151:dbl[], w7115:dbl[], w7113:dbl[], w7112:dbl[], w7110:dbl[], w7109:dbl[], w7108:dbl[], w7107:dbl[])
            n1393 = Divide(x=w7156, y=w7154) -> (x/y=w7137:dbl[])
            n1394 = Divide(x=w7155, y=w7154) -> (x/y=w7136:dbl[])
            n1395 = Divide(x=w7153, y=w7151) -> (x/y=w7135:dbl[])
            n1396 = Divide(x=w7152, y=w7151) -> (x/y=w7134:dbl[])
            n1397 = Divide(x=w7115, y=w7113) -> (x/y=w7114:dbl[])
            n1398 = Divide(x=w7112, y=w7110) -> (x/y=w7111:dbl[])
            n1399 = Bundle("T1 Y", "T1 X", "T1 Sum", "T2 Y", "T2 X", "T2 Sum", "T1 FB X", "T2 FB Sum", "T2 FB X", "T2 FB Sum", "PSD Y", "PSD X", "PSD Sum") -> (w7138:T46)  [unwired: 1 out]
            n1400 = Build Array(w7137, w7136, w7154, w7135, w7134, w7151, w7114, w7113, w7111, w7110, w7109, w7108, w7107) -> (w7106:dbl[][])
            n1401 = Cluster To Array(cluster=w7138) -> (array=w7129:string[])
          }
          frame "IR-QPD + PSD + FB-QPD XY positions" {
            w7215 = 4  # Channel pattern
            # "time average x2 the 3 psd signals (detection laser)"
            # "deinterlace 3 signals from qpds"
            n1402 = Decimate 1D Array(w7239) -> (w7238:i16[], w7237:i16[], w7216:i16[], w7236:i16[], w7182:i16[], w7228:i16[], w7227:i16[], w7204:i16[])
            n1403 = Decimate 1D Array "QPD Y"(w7238) -> (w7235:i16[], w7218:i16[])
            n1404 = call "downsample 1D array - double.vi"("Ave N"=2.0, "Array In"=w7228) -> ("Array Out"=w7203:dbl[])  [unwired: 1 out]
            n1405 = call "downsample 1D array - double.vi"("Ave N"=2.0, "Array In"=w7227) -> ("Array Out"=w7202:dbl[])  [unwired: 1 out]
            n1406 = Decimate 1D Array "Feedback Sum"(w7216) -> (w7200:i16[], w7198:i16[])
            n1407 = Decimate 1D Array "Feedback Y"(w7182) -> (w7181:i16[], w7180:i16[])
            n1408 = Decimate 1D Array "Feedback X"(w7204) -> (w7201:i16[], w7199:i16[])
            n1409 = Decimate 1D Array "QPD Sum"(w7236) -> (w7233:i16[], w7231:i16[])
            n1410 = Decimate 1D Array "QPD X"(w7237) -> (w7234:i16[], w7232:i16[])
            n1411 = Interleave 1D Arrays(w7235, w7234, w7233, w7218, w7232, w7231, w7181, w7201, w7200, w7180, w7199, w7198, w7203, w7202) -> (w7226:dbl[])
            n1412 = To Word Integer(number=w7226) -> (16bit integer=w7170:i16[])
            n1413 = Divide(x=w7226, y=3276.7) -> (x/y=w7225:dbl[])
            n1414 = Decimate 1D Array(w7225) -> (w7224:dbl[], w7223:dbl[], w7222:dbl[], w7221:dbl[], w7220:dbl[], w7219:dbl[], w7177:dbl[], w7191:dbl[], w7175:dbl[], w7176:dbl[], w7189:dbl[], w7173:dbl[], w7187:dbl[], w7185:dbl[])
            n1415 = Divide(x=w7224, y=w7222) -> (x/y=w7208:dbl[])
            n1416 = Divide(x=w7223, y=w7222) -> (x/y=w7207:dbl[])
            n1417 = Divide(x=w7221, y=w7219) -> (x/y=w7206:dbl[])
            n1418 = Divide(x=w7220, y=w7219) -> (x/y=w7205:dbl[])
            n1419 = Divide(x=w7177, y=w7175) -> (x/y=w7174:dbl[])
            n1420 = Divide(x=w7191, y=w7175) -> (x/y=w7190:dbl[])
            n1421 = Divide(x=w7176, y=w7173) -> (x/y=w7172:dbl[])
            n1422 = Divide(x=w7189, y=w7173) -> (x/y=w7188:dbl[])
            n1423 = Negate(x=w7185) -> (-x=w7183:dbl[])
            n1424 = Divide(x=w7187, y=w7183) -> (x/y=w7186:dbl[])
            n1425 = Bundle("T1 Y", "T1 X", "T1 Sum", "T2 Y", "T2 X", "T2 Sum", "T1 FB Y", "T1 FB X", "T1 FB Sum", "T2 FB Y", "T2 FB X", "T2 FB Sum", "PSD X", "PSD Y Sum") -> (w7171:T47)  [unwired: 1 out]
            n1426 = Build Array(w7208, w7207, w7222, w7206, w7205, w7219, w7174, w7190, w7175, w7172, w7188, w7173, w7186, w7185) -> (w7184:dbl[][])
            n1427 = Cluster To Array(cluster=w7171) -> (array=w7217:string[])
          }
        }
      }
    }
    "AI labels" <- w5508
    n1428 = Decimate 1D Array(w5478) -> (w5506:u32[], w5442:u32[])
    n1429 = local read "DMA Update Period (s)"() -> (w5517:dbl)
    n1430 = local read "BD 1 Frequency 2 (MHz)"() -> (w5384:dbl)
    n1431 = local read "BD 1 Frequency 1 (MHz)"() -> (w5385:dbl)
    n1432 = Build Array(w5506, w5442) -> (w5585:u32[][])
    n1433 = local read "Data Period (s)"() -> (w5491:dbl)
    n1434 = Decimate 1D Array(w5392) -> (w5415:i16[], w5414:i16[], w5412:i16[], w5411:i16[])  [unwired: 9 out]
    n1435 = To Double Precision Float(number=w5585) -> (double precision float=w5586:dbl[][])
    n1436 = local read "APD Integration Time (s)"() -> (w5455:dbl)
    n1437 = Divide(x=w5415, y=w5414) -> (x/y=w5416:dbl[])
    n1438 = Divide(x=w5412, y=w5411) -> (x/y=w5413:dbl[])
    n1439 = feedback #1(0.0) -> (w5429:dbl)
    n1440 = Add(x=w5517, y=w5429) -> (x+y=w5625:dbl)
    n1441 = feedback-in #1(w5625) -> ()
    n1442 = local read "AOM X Cal (nm/MHz)"() -> (w5382:dbl)
    n1443 = To Time Stamp(1:w5429) -> (0:w5428:timestamp)
    n1444 = Split 1D Array(array=w5416, index="N El. to Ave.") -> (second subarray=w5419:dbl[])  [unwired: 1 out]
    n1445 = Split 1D Array(array=w5413, index="N El. to Ave.") -> (second subarray=w5418:dbl[])  [unwired: 1 out]
    n1446 = local read "Trap X AI1 (DMA)"() -> (w5417:T13)
    n1447 = Multiply(x=w5491, y="Trap Disp. Downsample") -> (x*y=w5430:dbl)
    "Display Period (s)" <- w5430
    n1448 = Bundle("BD 1 Frequency 1 (MHz)"=w5385, "BD 1 Frequency 2 (MHz)"=w5384) -> (w5386:T48)  [unwired: 1 out]
    n1449 = for "Trap AI" {
      tunnel: [w6905] -> w5619 mode=indexing
      tunnel: w5428 -> [w6895]
      tunnel: "Trap Disp. Downsample" -> [w6903]
      tunnel: w5509 -> [w6901] mode=indexing
      tunnel: w5491 -> [w6900]
      tunnel: w5508 -> [w6899] mode=indexing
      tunnel: w5427 -> [w6898]
      tunnel: [w6897] -> w5466 mode=indexing
      tunnel: w5430 -> [w6896]
      n1450 = Bundle By Name("Y"=w6901, "dt"=w6900) -> (w6902:waveform(dbl))  [unwired: 1 out]
      n1451 = Set Waveform Attribute(5:w6899, 6:w6898, 7:w6902) -> (3:w6897:waveform(dbl))  [unwired: 1 in, 2 out]
      n1452 = call "downsample 1D array - double.vi"("Ave N"=w6903, "Array In"=w6901) -> ("Array Out"=w6904:dbl[])  [unwired: 1 out]
      n1453 = Bundle By Name(cluster=w6897, "t0"=w6895, "Y"=w6904, "dt"=w6896) -> (w6905:waveform(dbl))
    }
    n1454 = call <vilib>:"Mean.vi"("X"=w5418) -> ("mean"=w5406:dbl)  [unwired: 1 out]
    n1455 = call <vilib>:"Mean.vi"("X"=w5419) -> ("mean"=w5407:dbl)  [unwired: 1 out]
    n1456 = Cluster To Array(cluster=w5386) -> (array=w5383:dbl[])
    n1457 = Reciprocal(x=w5430) -> (1/x=→"Trap Disp. Freq. (Hz)":dbl)
    n1458 = local read "Data points/scans (MCL)"() -> (w5597:dbl)
    n1459 = To Fixed-Point(number=w5406) -> (fixed-point=w5404:fxp<+/-,16,1>)  [unwired: 1 in]
    n1460 = To Fixed-Point(number=w5407) -> (fixed-point=w5405:fxp<+/-,16,1>)  [unwired: 1 in]
    n1461 = Bundle("Trap 1 Pos.", "Trap 2 Pos.") -> (w5426:cluster{string, string})  [unwired: 1 out]
    n1462 = Bundle By Name(cluster=w5417, "Set 1"=w5405, "Set 2"=w5404) -> (→"Trap X AI1 (DMA)":T13)
    n1463 = Cluster To Array(cluster=w5426) -> (array=w5423:string[])
    n1464 = for "Trap Position" {
      tunnel: w5432 -> [w5882] mode=indexing
      tunnel: "Trap Disp. Downsample" -> [w5881]
      tunnel: w5430 -> [w5879]
      tunnel: w5428 -> [w5878]
      tunnel: w5427 -> [w5876]
      tunnel: w5423 -> [w5875] mode=indexing
      tunnel: [w5874] -> w5381 mode=indexing
      tunnel: w5383 -> [w5872] mode=indexing
      tunnel: w5382 -> [w5870]
      n1465 = call "downsample 1D array - double.vi"("Ave N"=w5881, "Array In"=w5882) -> ("Array Out"=w5880:dbl[])  [unwired: 1 out]
      n1466 = Subtract(x=w5880, y=w5872) -> (x-y=w5873:dbl[])
      n1467 = Multiply(x=w5870, y=w5873) -> (x*y=w5871:dbl[])
      n1468 = Bundle By Name("Y"=w5871, "dt"=w5879, "t0"=w5878) -> (w5877:waveform(dbl))  [unwired: 1 out]
      n1469 = Set Waveform Attribute(5:w5875, 6:w5876, 7:w5877) -> (3:w5874:waveform(dbl))  [unwired: 1 in, 2 out]
    }
    "Trap Positions" <- w5381
    n1470 = Bundle("APD 1", "APD 2") -> (w5618:cluster{string, string})  [unwired: 1 out]
    n1471 = Cluster To Array(cluster=w5618) -> (array=w5615:string[])
    n1472 = for "APD" {
      tunnel: w5586 -> [w6884] mode=indexing
      tunnel: w5455 -> [w6892]
      tunnel: [w6888] -> w5462 mode=indexing
      tunnel: "APD Disp. Scale" -> [w6889]
      tunnel: w5427 -> [w6887]
      tunnel: w5615 -> [w6886] mode=indexing
      tunnel: "APD Disp. Downsample" -> [w6882]
      tunnel: [w6885] -> w5614
      tunnel: w5428 -> [w6881]
      n1473 = call "integrate 1D array interval - double.vi"("Ave N"=w6882, "Array In"=w6884) -> ("Array Out"=w6883:dbl[])  [unwired: 1 out]
      n1474 = Multiply(x=w6892, y=w6882) -> (x*y=w6885:dbl)
      n1475 = Divide(x=w6883, y=w6889) -> (x/y=w6890:dbl[])
      n1476 = Bundle By Name("t0"=w6881, "Y"=w6890, "dt"=w6885) -> (w6891:waveform(dbl))  [unwired: 1 out]
      n1477 = Set Waveform Attribute(5:w6886, 6:w6887, 7:w6891) -> (3:w6888:waveform(dbl))  [unwired: 1 in, 2 out]
    }
    "APD Display Period (s)" <- w5614
    n1478 = Reciprocal(x=w5614) -> (1/x=→"APD Display Freq. (Hz)":dbl)
    n1479 = local read "Display Period (s)"() -> (w5490:dbl)
    n1480 = Increment(x=w5597) -> (x+1=w5598:dbl)
    n1481 = Index Array(array=w5381, index=0) -> (element=w5379:waveform(dbl))
    n1482 = To Double Precision Float(number=w5506) -> (double precision float=w5505:dbl[])
    n1483 = feedback #2(w5598) -> (w5601:dbl)
    n1484 = Select(t=0, s=w5588, f=w5601) -> (s? t:f=w5594:dbl)
    n1485 = Array Size(array=w5505) -> (size(s)=w5600:i32)
    n1486 = Add(x=w5600, y=w5594) -> (x+y=w5595:dbl)
    n1487 = Unbundle By Name(w5379) -> ("Y"=w5377:dbl[])
    n1488 = feedback #3(w5506) -> (w5584:u32[])
    n1489 = Build Array (concatenate)(w5584, w5506) -> (w5581:u32[])
    n1490 = feedback #4(w5442) -> (w5461:u32[])
    n1491 = Divide(x="Bead Sep. Int. Time (s)", y=w5490) -> (x/y=w5375:dbl)
    n1492 = Build Array (concatenate)(w5461, w5442) -> (w5460:u32[])
    n1493 = Greater?(x=w5595, y=w5597) -> (0:w5596:bool)
    n1494 = feedback #5(w5377) -> (w5378:dbl[])
    n1495 = Build Array (concatenate)(w5377, w5378) -> (w5376:dbl[])
    n1496 = Select(t=w5594, s=w5596, f=w5595) -> (s? t:f=w5593:dbl)
    n1497 = feedback-in #2(w5593) -> ()
    n1498 = Array Size(array=w5581) -> (size(s)=w5578:i32)
    n1499 = Array Size(array=w5506) -> (size(s)=w5580:i32)
    n1500 = local read "MCL Scanning"() -> (w5591:bool)
    n1501 = local read "APD Integration Time (s)"() -> (w5469:dbl)
    n1502 = Build Array (concatenate)(w5462, w5619) -> (w5464:waveform(dbl)[])
    "All Signals" <- w5464
    n1503 = Split 1D Array(array=w5376, index=w5375) -> (first subarray=w5369:dbl[])  [unwired: 1 out]
    n1504 = feedback-in #5(w5369) -> ()
    n1505 = Multiply(x=w5580, y="APD Ave N") -> (x*y=w5579:dbl)
    n1506 = Greater?(x=w5578, y=w5579) -> (0:w5582:bool)
    n1507 = Not(x=w5596) -> (.not. x?=w5590:bool)
    n1508 = To Double Precision Float(number=w5442) -> (double precision float=w5441:dbl[])
    n1509 = call <vilib>:"Mean.vi"("X"=w5369) -> ("mean"=w5368:dbl)  [unwired: 1 out]
    "Mean T1 Position (nm)" <- w5368
    n1510 = Subtract(x=w5369, y=w5368) -> (x-y=w5374:dbl[])
    n1511 = Square(x=w5374) -> (x^2=w5373:dbl[])
    n1512 = And(x=w5590, y=w5591) -> (x .and. y?=w5592:bool)
    n1513 = call <vilib>:"Mean.vi"("X"=w5373) -> ("mean"=w5372:dbl)  [unwired: 1 out]
    n1514 = case shown="True" w5582 {
      tunnel: w5581 -> [w6465 w6472]
      tunnel: [w6465 w6470] -> w5522
      tunnel: w5579 -> [_ w6467]
      tunnel: w5578 -> [_ w6471]
      tunnel: w5460 -> [w6464 w6469]
      tunnel: [w6464 w6466] -> w5457
      frame False {
      }
      frame True {
        n1515 = Subtract(x=w6471, y=w6467) -> (x-y=w6468:dbl)
        n1516 = Array Subset(array=w6472, index=w6468, length=w6467) -> (w6470:u32[])
        n1517 = Array Subset(array=w6469, index=w6468, length=w6467) -> (w6466:u32[])
      }
    }
    n1518 = feedback-in #3(w5522) -> ()
    n1519 = feedback-in #4(w5457) -> ()
    n1520 = Or(x=w5592, y=w5588) -> (x .or. y?=w5589:bool)
    n1521 = Square Root(x=w5372) -> (sqrt(x)=w5371:dbl)
    n1522 = Equal?(x="Tab Control 6", y=T37."High Res Display") -> (x = y?=w5512:bool)
    n1523 = Multiply(x="APD Disp. Scale", y=w5462) -> (x*y=w5471:waveform(dbl)[])
    n1524 = Multiply(x="APD Disp. Downsample", y=w5469) -> (x*y=w5467:dbl)